vi "UHR-Fleezers Control (host) - 12.7e.vi"() -> ()   [LabVIEW 2012] (continued)
                  frame #11 {
                    n1316 = property on="Load parameters" class="Bool (strict)"("Val(Sgnl)"=TRUE ("Value (Signaling)")) -> ()  [unwired: 2 in, 2 out]
                  }
                }
              }
            }
          }
          frame #9 {
            n1317 = property on="Read Cal" class="Bool (strict)"("Val(Sgnl)"=TRUE ("Value (Signaling)")) -> ()  [unwired: 2 in, 2 out]
          }
          frame #10 {
            n1318 = Wait (ms)(milliseconds to wait=u32 1000) -> ()  [unwired: 1 out]
          }
          frame #11 {
            n1319 = property on="Fish for Tether" class="Bool (strict)"("Val(Sgnl)"=TRUE ("Value (Signaling)")) -> ()  [unwired: 2 in, 2 out]
          }
        }
        n1320 = local write "Cal/Data Acq. Spot"(FALSE ("Cal/Data Acq. Spot")) -> ()
      }
      event "Dump Beads": Value Change {
        n1321 = event-data() -> ()  [unwired: 1 in, 5 out]
        n1322 = flat-sequence {
          tunnel: ["Dump spot flow on?"] -> w1951
          tunnel: [w1962] -> w1952
          tunnel: w1951 -> [w1962]
          tunnel: w1955 -> [w1967]
          tunnel: w1954 -> [w1966]
          tunnel: [w1964] -> w1953
          tunnel: w1952 -> [w1964]
          tunnel: w1953 -> [w1977]
          frame #0 {
            w1956 = FALSE ("Value (Signaling)")
            n1323 = local read "Saving..."() -> (w1958:bool)
            n1324 = local write "Dump Beads"(FALSE ("Dump Beads")) -> ()
            n1325 = property on="Inject Pump 3" class="Bool (strict)"("Val(Sgnl)"=w1956) -> ()  [unwired: 2 in, 2 out]
            n1326 = property on="Inject Pump 1" class="Bool (strict)"("Val(Sgnl)"=w1956) -> ()  [unwired: 2 in, 2 out]
            n1327 = local write "Stop Saving"(w1958) -> ()
          }
          frame #1 {
            w1959 = FALSE ("Fl. Triggered...")
            n1328 = case shown="True" "Dump spot flow on?" {
              frame False {
              }
              frame True {
                n1329 = property on="Sample Channel\nFlow" class="Bool (strict)"("Val(Sgnl)"=TRUE ("Stage Moving")) -> ()  [unwired: 2 in, 2 out]
              }
            }
            n1330 = local write "Fl. Triggered..."(w1959) -> ()
            n1331 = local write "Tether"(w1959) -> ()
            n1332 = property on="Green Laser ON" class="Bool (strict)"("Val(Sgnl)"=w1959) -> ()  [unwired: 2 in, 2 out]
            n1333 = property on="Trap Pos. FB ON" class="Bool (strict)"("Val(Sgnl)"=w1959) -> ()  [unwired: 2 in, 2 out]
            n1334 = property on="Trap Trig. Fl." class="Bool (strict)"("Val(Sgnl)"=w1959) -> ()  [unwired: 2 in, 2 out]
            n1335 = property on="Fl. Triggered..." class="Bool (strict)"("Val(Sgnl)"=w1959) -> ()  [unwired: 2 in, 2 out]
            n1336 = property on="Dip for Protein" class="Bool (strict)"("Val(Sgnl)"=w1959) -> ()  [unwired: 2 in, 2 out]
            n1337 = property on="Pause dwell" class="Bool (strict)"("Val(Sgnl)"=w1959) -> ()  [unwired: 2 in, 2 out]
          }
          frame #2 {
            n1338 = property on="Trap Pos. FB Offset Factor" class="DigNum (strict)"("Val(Sgnl)"=i64 0 ("Value (Signaling)")) -> ()  [unwired: 2 in, 2 out]
          }
          frame #3 {
            n1339 = local read "Saved Stage Positions"() -> (w1968:dbl[][])
            n1340 = local write "Stage Moving"(TRUE ("Stage Moving")) -> ()
            n1341 = Array Subset(array=w1968, index (row)=3 ("index"), length (row)=1 ("length"), index (col)=1 ("index"), length (col)=3 ("length")) -> (w1973:dbl[][])
            n1342 = Reshape Array(w1973, 3 ("dimension size")) -> (w1971:dbl[])
            n1343 = Array To Cluster(array=w1971) -> (cluster=w1970:cluster{"[0]":dbl, "[1]":dbl, "[2]":dbl})
            n1344 = call "Set Stage Position.vi"("Position"=w1970, "error in"=w1966, "VISA resource name in"=w1967) -> ()  [unwired: 3 out]
          }
          frame #4 {
            w1978 = FALSE ("Value (Signaling)")
            n1345 = case shown="True" w1977 {
              frame False {
              }
              frame True {
                n1346 = property on="Sample Channel\nFlow" class="Bool (strict)"("Val(Sgnl)"=FALSE ("Stage Moving")) -> ()  [unwired: 2 in, 2 out]
              }
            }
            n1347 = property on="Trap 1 (ON/OFF)" class="Bool (strict)"("Val(Sgnl)"=w1978) -> ()  [unwired: 2 in, 2 out]
            n1348 = property on="Trap 2 (ON/OFF)" class="Bool (strict)"("Val(Sgnl)"=w1978) -> ()  [unwired: 2 in, 2 out]
            n1349 = call <vilib>:"Beep.vi"() -> ()  [unwired: 3 in, 9 out]
          }
          frame #5 {
            n1350 = property on="Move Cap. 2 (ADig Top)" class="Bool (strict)"("Val(Sgnl)"=TRUE ("Value (Signaling)")) -> ()  [unwired: 2 in, 2 out]
            n1351 = property on="Tab Control" class="TabCtl (strict)"("Val(Sgnl)"=T31."Status" ("Value (Signaling)")) -> ()  [unwired: 2 in, 2 out]
          }
        }
      }
      event "Dip for Protein": Value Change {
        n1352 = event-data() -> ()  [unwired: 1 in, 5 out]
        n1353 = case shown="True" "Dip for Protein" {
          tunnel: w1984 -> [_ w1986]
          tunnel: w1983 -> [_ w1985]
          frame False {
          }
          frame True {
            n1354 = while {
              tunnel: w1986 -> [w1997]
              tunnel: w1985 -> [w1996]
              i -> [w1991]
              stop <- w1993 stop-if-true
              n1355 = Increment(x=w1991) -> (x+1=→"Dip #":i32)
              n1356 = flat-sequence {
                tunnel: w1996 -> [w2008]
                tunnel: w1997 -> [w2009]
                tunnel: [w2009] -> w2001
                tunnel: [w2008] -> w2000
                tunnel: [w2002] -> w1987
                tunnel: [w2014] -> w1995
                tunnel: [w2015] -> w1994
                tunnel: w2001 -> [w2016]
                tunnel: w2000 -> [w2017]
                tunnel: [w2012] -> w1988
                tunnel: w1987 -> [w2012]
                tunnel: [w2025] -> w1999
                tunnel: w1995 -> [w2025]
                tunnel: [w2024] -> w1998
                tunnel: w1994 -> [w2024]
                tunnel: [w2021] -> w1992
                tunnel: [w2020] -> w1989
                tunnel: w1988 -> [w2020]
                tunnel: w1998 -> [w2045]
                tunnel: w1999 -> [w2046]
                tunnel: w1992 -> [w2047]
                tunnel: w1989 -> [w2044]
                tunnel: [w2103] -> w1993
                frame #0 {
                  n1357 = local read "Trap Pos. FB ON"() -> (w2002:bool)
                  n1358 = Compound Arithmetic op=AND("Flow ON\nduring dip?", "FB OFF when \nflow ON", w2002) -> (w2003:bool)
                  n1359 = case shown="True" "Move trap \nbefore dip move?" {
                    frame False {
                    }
                    frame True {
                      n1360 = property on="Trap Delta (MHz)" class="DigNum (strict)"("Val(Sgnl)"="Dipping Delta (MHz)") -> ()  [unwired: 2 in, 2 out]
                    }
                  }
                  n1361 = property on="Green Laser ON" class="Bool (strict)"("Val(Sgnl)"="Green ON\nbefore dip?") -> ()  [unwired: 2 in, 2 out]
                  n1362 = property on="Sample Channel\nFlow" class="Bool (strict)"("Val(Sgnl)"="Flow ON\nduring dip?") -> ()  [unwired: 2 in, 2 out]
                  n1363 = case shown="True" w2003 {
                    frame False {
                    }
                    frame True {
                      n1364 = property on="Trap Pos. FB ON" class="Bool (strict)"("Val(Sgnl)"=FALSE ("Value (Signaling)")) -> ()  [unwired: 2 in, 2 out]
                    }
                  }
                }
                frame #1 {
                  n1365 = local read "Saved Stage Positions"() -> (w2019:dbl[][])
                  n1366 = local write "Cancel dwell"(FALSE ("Cancel dwell")) -> ()
                  n1367 = call "move to saved stage position.vi"("error in"=w2017, "Stage VISA resource name in"=w2016, "Position"="Dip Stage \nPosition", "Saved Stage Positions"=w2019) -> ("VISA resource name out"=w2014:refnum<visa-resource-name>, "error out"=w2015:errorcluster)
                }
                frame #2 {
                  n1368 = node-c288() -> (w2023:T23)  [unwired: 4 in]
                  n1369 = timed-loop {
                    timing: w2023 -> [_]
                    timing-out: [_] -> w2022
                    tunnel: [w2029] -> w2021
                    i -> [w2026]
                    stop <- w2030 stop-if-true
                    n1370 = node-c288() -> ()  [unwired: 1 in, 1 out]
                    n1371 = Greater Or Equal?(x=w2026, y="Dip Duration (s)") -> (x >= y?=w2038:bool)
                    n1372 = local read "Dip for Protein"() -> (w2031:bool)
                    n1373 = local read "Dump Beads"() -> (w2028:bool)
                    n1374 = local read "Cancel dwell"() -> (w2037:bool)
                    n1375 = local read "Pause dwell"() -> (w2034:bool)
                    n1376 = Not(x=w2031) -> (.not. x?=w2036:bool)
                    n1377 = Compound Arithmetic op=OR(w2037, w2038, w2036) -> (w2035:bool)
                    n1378 = Select(t=FALSE, s=w2034, f=w2035) -> (s? t:f=w2032:bool)
                    n1379 = Not(x=w2028) -> (.not. x?=w2027:bool)
                    n1380 = node-c288() -> ()  [unwired: 1 in, 1 out]
                    n1381 = And(x=w2031, y=w2027) -> (x .and. y?=w2029:bool)
                    n1382 = Or(x=w2032, y=w2028) -> (x .or. y?=w2030:bool)
                    "Dip Time (s)" <- w2026
                  }
                  n1383 = node-c288(w2022) -> ()  [unwired: 1 out]
                }
                frame #3 {
                  n1384 = case shown="True" w2047 {
                    tunnel: w2046 -> [_ w2052]
                    tunnel: w2045 -> [_ w2051]
                    tunnel: w2044 -> [_ w2048]
                    frame False {
                    }
                    frame True {
                      n1385 = flat-sequence {
                        tunnel: w2051 -> [w2056]
                        tunnel: w2052 -> [w2057]
                        tunnel: [w2057] -> w2050
                        tunnel: [w2056] -> w2049
                        tunnel: w2048 -> [w2053]
                        tunnel: w2050 -> [w2067]
                        tunnel: w2049 -> [w2066]
                        tunnel: w2048 -> [w2075]
                        frame #0 {
                          n1386 = local read "Sample Channel\nFlow"() -> (w2055:bool)
                          n1387 = case shown="True" w2055 {
                            tunnel: "Flow ON \nduring return\nfrom dip?" -> [w2058 w2061]
                            tunnel: w2053 -> [_ w2060]
                            frame False {
                              n1388 = case shown="True" w2058 {
                                frame False {
                                }
                                frame True {
                                n1389 = property on="Sample Channel\nFlow" class="Bool (strict)"("Val(Sgnl)"=TRUE ("Value (Signaling)")) -> ()  [unwired: 2 in, 2 out]
                                }
                              }
                            }
                            frame True {
                              n1390 = case shown="False" w2061 {
                                tunnel: w2060 -> [w2062 _]
                                frame False {
                                n1391 = property on="Trap Pos. FB ON" class="Bool (strict)"("Val(Sgnl)"=w2062) -> ()  [unwired: 2 in, 2 out]
                                n1392 = property on="Sample Channel\nFlow" class="Bool (strict)"("Val(Sgnl)"=FALSE ("Value (Signaling)")) -> ()  [unwired: 2 in, 2 out]
                                }
                                frame True {
                                }
                              }
                            }
                          }
                        }
                        frame #1 {
                          # "For turning on green laser before stage reaches lower spot"
                          n1393 = case shown="True" "Green ON\nafter start\nreturn?" {
                            frame False {
                            }
                            frame True {
                              n1394 = flat-sequence {
                                frame #0 {
                                n1395 = Multiply(x="Green delay after \nstart return (s)", y=1000.0) -> (x*y=w2072:dbl)
                                n1396 = Wait (ms)(milliseconds to wait=w2072) -> ()  [unwired: 1 out]
                                }
                                frame #1 {
                                n1397 = property on="Green Laser ON" class="Bool (strict)"("Val(Sgnl)"=TRUE ("Value (Signaling)")) -> ()  [unwired: 2 in, 2 out]
                                }
                              }
                            }
                          }
                          n1398 = local read "Saved Stage Positions"() -> (w2070:dbl[][])
                          n1399 = local write "Cancel dwell"(FALSE ("Cancel dwell")) -> ()
                          n1400 = call "move to saved stage position.vi"("error in"=w2066, "Stage VISA resource name in"=w2067, "Position"="Return Stage \nPosition", "Saved Stage Positions"=w2070) -> ("error out"=w2068:errorcluster)  [unwired: 1 out]
                          n1401 = local write "Stage Control Serial Error"(w2068) -> ()
                        }
                        frame #2 {
                          n1402 = property on="Trap Pos. FB ON" class="Bool (strict)"("Val(Sgnl)"=w2075) -> ()  [unwired: 2 in, 2 out]
                          n1403 = case shown="True" "Green ON \nafter return?" {
                            frame False {
                            }
                            frame True {
                              n1404 = property on="Green Laser ON" class="Bool (strict)"("Val(Sgnl)"=TRUE ("Value (Signaling)")) -> ()  [unwired: 2 in, 2 out]
                            }
                          }
                          n1405 = case shown="True" "Move trap after return?" {
                            frame False {
                            }
                            frame True {
                              n1406 = property on="Trap Delta (MHz)" class="DigNum (strict)"("Val(Sgnl)"="Dip Trap Delta 2 (MHz)") -> ()  [unwired: 2 in, 2 out]
                            }
                          }
                          n1407 = case shown="True" "Save data after return?" {
                            frame False {
                            }
                            frame True {
                              n1408 = property on="Start Saving" class="Bool (strict)"("Val(Sgnl)"=TRUE ("Value (Signaling)")) -> ()  [unwired: 2 in, 2 out]
                            }
                          }
                          n1409 = property on="Sample Channel\nFlow" class="Bool (strict)"("Val(Sgnl)"="Flow ON\nduring daq?") -> ()  [unwired: 2 in, 2 out]
                        }
                        frame #3 {
                          n1410 = node-c288() -> (w2084:T23)  [unwired: 4 in]
                          n1411 = timed-loop {
                            timing: w2084 -> [_]
                            timing-out: [_] -> w2083
                            i -> [w2085]
                            stop <- w2087 stop-if-true
                            n1412 = node-c288() -> ()  [unwired: 1 in, 1 out]
                            n1413 = local read "Dump Beads"() -> (w2086:bool)
                            n1414 = Greater Or Equal?(x=w2085, y="Dwell Duration (s)") -> (x >= y?=w2092:bool)
                            n1415 = local read "Dip for Protein"() -> (w2089:bool)
                            n1416 = Not(x=w2089) -> (.not. x?=w2088:bool)
                            n1417 = Compound Arithmetic op=OR(w2092, "Cancel dwell", w2088) -> (w2091:bool)
                            n1418 = node-c288() -> ()  [unwired: 1 in, 1 out]
                            n1419 = Select(t=FALSE, s="Pause dwell", f=w2091) -> (s? t:f=w2094:bool)
                            n1420 = Or(x=w2094, y=w2086) -> (x .or. y?=w2087:bool)
                            "Dwell Time (s)" <- w2085
                          }
                          n1421 = node-c288(w2083) -> ()  [unwired: 1 out]
                        }
                      }
                    }
                  }
                }
                frame #4 {
                  n1422 = local read "Dip for Protein"() -> (w2104:bool)
                  n1423 = local read "Dump Beads"() -> (w2101:bool)
                  n1424 = local write "Cancel dwell"(FALSE ("Cancel dwell")) -> ()
                  n1425 = Not(x=w2104) -> (.not. x?=w2105:bool)
                  n1426 = Not(x="Cont. Repeat Dipping?") -> (.not. x?=w2107:bool)
                  n1427 = Compound Arithmetic op=OR(w2105, w2107, w2101) -> (w2103:bool)
                }
              }
            }
          }
        }
      }
      event "Profile": Value Change {
        n1428 = event-data() -> ()  [unwired: 1 in, 5 out]
        n1429 = flat-sequence {
          tunnel: w2116 -> [w2119]
          tunnel: w2115 -> [w2127]
          tunnel: [w2121] -> w2114
          tunnel: [w2120] -> w2113
          tunnel: [w2118] -> w2111
          tunnel: [w2117] -> w2108
          tunnel: w2114 -> [w2134]
          tunnel: w2113 -> [w2133]
          tunnel: [w2131] -> w2112
          tunnel: w2111 -> [w2132]
          tunnel: [w2130] -> w2110
          tunnel: [w2129] -> w2109
          tunnel: w2108 -> [w2129]
          tunnel: w2112 -> [w2138]
          tunnel: w2110 -> [w2137]
          tunnel: w2109 -> [w2136]
          frame #0 {
            n1430 = call "Read Stage Position.vi"("error in"=w2127, "VISA resource name in"=w2119) -> ("Current Position"=w2117:cluster{dbl, dbl, dbl}, "error out"=w2120:errorcluster, "VISA resource name out"=w2118:refnum<visa-resource-name>)  [unwired: 1 out]
            "Current Position" <- w2117
            n1431 = local write "Stage Control Serial Error"(w2120) -> ()
            n1432 = Unbundle(w2117) -> (w2124:dbl, w2126:dbl, w2122:dbl)
            n1433 = Add(x=w2126, y="Y change (mm)") -> (x+y=w2123:dbl)
            n1434 = Bundle(w2124, w2123, w2122) -> (w2121:cluster{dbl, dbl, dbl})  [unwired: 1 in]
          }
          frame #1 {
            # "move to new position and start saving"
            n1435 = local write "Stage Moving"(TRUE ("Stage Moving")) -> ()
            n1436 = local write "Start Saving"(TRUE ("Start Saving")) -> ()
            n1437 = call "Set Stage Position.vi"("Position"=w2134, "error in"=w2133, "VISA resource name in"=w2132) -> ("error out"=w2130:errorcluster, "VISA resource name out"=w2131:refnum<visa-resource-name>)  [unwired: 1 out]
          }
          frame #2 {
            # "go back to start"
            n1438 = call "Set Stage Position.vi"("Position"=w2136, "error in"=w2137, "VISA resource name in"=w2138) -> ()  [unwired: 3 out]
          }
          frame #3 {
            # "stop saving"
            n1439 = local write "Stop Saving"(TRUE ("Stop Saving")) -> ()
            n1440 = local write "Stage Moving"(FALSE ("Stage Moving")) -> ()
          }
        }
      }
      event "Move to Position 1", "Move to Position 2", "Move to Position 3", "Move to Position 4", "Move to Position 5", "Lower Ch. Cap.": Value Change {
        n1441 = event-data() -> ()  [unwired: 1 in, 5 out]
        n1442 = Or(x="Move to Position 5", y="Lower Ch. Cap.") -> (x .or. y?=w2144:bool)
        n1443 = Build Array("Move to Position 1", "Move to Position 2", "Move to Position 3", "Move to Position 4", w2144) -> (w2147:bool[])
        n1444 = Boolean Array To Number(Boolean array=w2147) -> (number=w2146:u32)
        n1445 = Logarithm Base 2(1:w2146) -> (0:w2145:dbl)
        n1446 = flat-sequence {
          tunnel: w2145 -> [w2156]
          tunnel: w2142 -> [w2154]
          tunnel: w2141 -> [w2153]
          frame #0 {
            n1447 = local read "Saved Stage Positions"() -> (w2164:dbl[][])
            n1448 = Array Subset(array=w2164, index (row)=w2156, length (row)=1 ("length"), index (col)=1 ("index"), length (col)=3 ("length")) -> (w2161:dbl[][])
            n1449 = Reshape Array(w2161, 3 ("dimension size")) -> (w2159:dbl[])
            n1450 = Array To Cluster(array=w2159) -> (cluster=w2158:cluster{"[0]":dbl, "[1]":dbl, "[2]":dbl})
            n1451 = call "Set Stage Position.vi"("Position"=w2158, "error in"=w2153, "VISA resource name in"=w2154) -> ("error out"=w2157:errorcluster)  [unwired: 2 out]
            n1452 = local write "Stage Moving"(TRUE ("Stage Moving")) -> ()
            n1453 = local write "Stage Control Serial Error"(w2157) -> ()
          }
          frame #1 {
            n1454 = local write "Stage Moving"(FALSE ("Stage Moving")) -> ()
            n1455 = call <vilib>:"Beep.vi"() -> ()  [unwired: 3 in, 9 out]
          }
        }
      }
      event "Got ADig bead": Value Change {
        n1456 = event-data() -> ()  [unwired: 1 in, 5 out]
        n1457 = flat-sequence {
          frame #0 {
            n1458 = local read "Cap 1 Samp Flow ON"() -> (w2168:bool)
            n1459 = case shown="True" w2168 {
              frame False {
              }
              frame True {
                n1460 = property on="Sample Channel\nFlow" class="Bool (strict)"("Val(Sgnl)"=TRUE ("Value (Signaling)")) -> ()  [unwired: 2 in, 2 out]
              }
            }
          }
          frame #1 {
            n1461 = property on="Inject Pump 3" class="Bool (strict)"("Val(Sgnl)"=FALSE ("Value (Signaling)")) -> ()  [unwired: 2 in, 2 out]
          }
          frame #2 {
            n1462 = property on="Move Cap. 1 (DNA Bottom)" class="Bool (strict)"("Val(Sgnl)"=TRUE ("Value (Signaling)")) -> ()  [unwired: 2 in, 2 out]
          }
        }
      }
      event "Force FB Data\nScript": Value Change {
        n1463 = event-data() -> ()  [unwired: 1 in, 5 out]
        n1464 = flat-sequence {
          tunnel: w2177 -> [w2181]
          tunnel: w2178 -> [w2182]
          tunnel: [w2182] -> w2173
          tunnel: [w2181] -> w2172
          tunnel: w2173 -> [w2185]
          tunnel: w2172 -> [w2184]
          tunnel: ["Trap Trig Fl."] -> w2174
          tunnel: [w2210] -> w2175
          tunnel: w2174 -> [w2210]
          tunnel: [w2214] -> w2176
          tunnel: w2175 -> [w2214]
          tunnel: w2176 -> [w2216]
          frame #0 {
            n1465 = property on="Trap Delta (MHz)" class="DigNum (strict)"("Val(Sgnl)"="Trap Delta Before Moving") -> ()  [unwired: 2 in, 2 out]
          }
          frame #1 {
            n1466 = local read "Saved Stage Positions"() -> (w2187:dbl[][])
            n1467 = local write "FB Trap Pos Offset"(0.0 ("FB Trap Pos Offset")) -> ()
            n1468 = property on="Trap Pos. FB Offset Factor" class="DigNum (strict)"("Val(Sgnl)"=i64 0 ("Value (Signaling)")) -> ()  [unwired: 2 in, 2 out]
            n1469 = local write "Stage Moving"(TRUE ("Stage Moving")) -> ()
            n1470 = call "move to saved stage position.vi"("error in"=w2184, "Stage VISA resource name in"=w2185, "Position"="Stage Position To Establish FB", "Saved Stage Positions"=w2187) -> ("error out"=w2183:errorcluster)  [unwired: 1 out]
            n1471 = local write "Stage Control Serial Error"(w2183) -> ()
          }
          frame #2 {
            n1472 = call <vilib>:"Beep.vi"() -> ()  [unwired: 3 in, 9 out]
            n1473 = Multiply(x="Wait (s)", y=u32 1000 ("milliseconds to wait")) -> (x*y=w2194:u32)
            n1474 = property on="Trap Delta (MHz)" class="DigNum (strict)"("Val(Sgnl)"="Starting \nTrap Delta (MHz)") -> ()  [unwired: 2 in, 2 out]
            n1475 = local write "Stage Moving"(FALSE ("Stage Moving")) -> ()
            n1476 = Wait (ms)(milliseconds to wait=w2194) -> ()  [unwired: 1 out]
            n1477 = property on="Tab Control 2" class="TabCtl (strict)"("Val(Sgnl)"=T6."Feedback on Trap Position" ("Value (Signaling)")) -> ()  [unwired: 2 in, 2 out]
            n1478 = property on="Tab Control" class="TabCtl (strict)"("Val(Sgnl)"=T32."Trap Control (RF)" ("Value (Signaling)")) -> ()  [unwired: 2 in, 2 out]
          }
          frame #3 {
            n1479 = property on="Set Reading to\nSetpoint" class="Bool (strict)"("Val(Sgnl)"=TRUE ("Value (Signaling)")) -> ()  [unwired: 2 in, 2 out]
            n1480 = Wait (ms)(milliseconds to wait=u32 500) -> ()  [unwired: 1 out]
          }
          frame #4 {
            n1481 = property on="Trap Pos. FB ON" class="Bool (strict)"("Val(Sgnl)"=TRUE ("Value (Signaling)")) -> ()  [unwired: 2 in, 2 out]
            n1482 = Wait (ms)(milliseconds to wait=u32 250) -> ()  [unwired: 1 out]
          }
          frame #5 {
            n1483 = case shown="False" "Trap Trig Fl." {
              frame False {
                n1484 = case shown="True" "Green ON after FB ON?" {
                  selector: "Green ON after FB ON?" -> [_ w2209]
                  frame False {
                  }
                  frame True {
                    n1485 = property on="Green Laser ON" class="Bool (strict)"("Val(Sgnl)"=w2209) -> ()  [unwired: 2 in, 2 out]
                  }
                }
              }
              frame True {
              }
            }
            n1486 = case shown="True" "Remove Action Offset" {
              tunnel: TRUE ("Value (Signaling)") -> [w2206 w2207]
              frame False {
                n1487 = property on="Remove Unwinding Offset" class="Bool (strict)"("Val(Sgnl)"=w2206) -> ()  [unwired: 2 in, 2 out]
              }
              frame True {
                n1488 = property on="Remove Action Offset" class="Bool (strict)"("Val(Sgnl)"=w2207) -> ()  [unwired: 2 in, 2 out]
              }
            }
            n1489 = Wait (ms)(milliseconds to wait=u32 250) -> ()  [unwired: 1 out]
          }
          frame #6 {
            n1490 = property on="Start Saving" class="Bool (strict)"("Val(Sgnl)"=TRUE ("Value (Signaling)")) -> ()  [unwired: 2 in, 2 out]
            n1491 = Wait (ms)(milliseconds to wait=u32 5000) -> ()  [unwired: 1 out]
          }
          frame #7 {
            w2213 = TRUE ("Value (Signaling)")
            n1492 = property on="Rem fb disp offset" class="Bool (strict)"("Val(Sgnl)"=w2213) -> ()  [unwired: 2 in, 2 out]
            n1493 = property on="Remove Offset" class="Bool (strict)"("Val(Sgnl)"=w2213) -> ()  [unwired: 2 in, 2 out]
            n1494 = Wait (ms)(milliseconds to wait=u32 100) -> ()  [unwired: 1 out]
          }
          frame #8 {
            n1495 = case shown="True" w2216 {
              frame False {
              }
              frame True {
                n1496 = local write "Trap Trig. Fl."(TRUE ("Value (Signaling)")) -> ()
              }
            }
          }
          frame #9 {
            n1497 = case shown="True" "Start dipping after?" {
              frame False {
              }
              frame True {
                n1498 = flat-sequence {
                  frame #0 {
                    n1499 = Multiply(x="Delay before dipping (s)", y=1000.0) -> (x*y=w2220:dbl)
                    n1500 = Wait (ms)(milliseconds to wait=w2220) -> ()  [unwired: 1 out]
                  }
                  frame #1 {
                    n1501 = property on="Dip for Protein" class="Bool (strict)"("Val(Sgnl)"=TRUE ("Value (Signaling)")) -> ()  [unwired: 2 in, 2 out]
                    n1502 = local write "Scripts"(T1."Dipping" ("Scripts")) -> ()
                  }
                }
              }
            }
          }
        }
      }
      event "Fixed Traps Data\nScript": Value Change {
        n1503 = event-data() -> ()  [unwired: 1 in, 5 out]
        n1504 = flat-sequence {
          frame #0 {
            n1505 = case shown="True" "Green ON" {
              frame False {
              }
              frame True {
                n1506 = property on="Green Laser ON" class="Bool (strict)"("Val(Sgnl)"=TRUE) -> ()  [unwired: 2 in, 2 out]
              }
            }
            n1507 = local write "Offset (nm)"(0.0 ("Offset (nm)")) -> ()
            n1508 = property on="Sample Channel\nFlow" class="Bool (strict)"("Val(Sgnl)"=FALSE ("Value (Signaling)")) -> ()  [unwired: 2 in, 2 out]
            n1509 = property on="Trap Delta (MHz)" class="DigNum (strict)"("Val(Sgnl)"="Fixed Traps Trap Delta (MHz)") -> ()  [unwired: 2 in, 2 out]
          }
          frame #1 {
            n1510 = Wait (ms)(milliseconds to wait=u32 1000) -> ()  [unwired: 1 out]
          }
          frame #2 {
            n1511 = local write "Start Saving"(TRUE ("Start Saving")) -> ()
          }
          frame #3 {
            n1512 = local read "Bead Sep. Int. Time (s)"() -> (w2231:dbl)
            n1513 = Multiply(x=w2231, y=1000.0) -> (x*y=w2233:dbl)
            n1514 = Wait (ms)(milliseconds to wait=w2233) -> ()  [unwired: 1 out]
          }
          frame #4 {
            n1515 = property on="Remove Offset" class="Bool (strict)"("Val(Sgnl)"=TRUE ("Value (Signaling)")) -> ()  [unwired: 2 in, 2 out]
          }
          frame #5 {
            n1516 = property on="Dip for Protein" class="Bool (strict)"("Val(Sgnl)"="Start dipping after?") -> ()  [unwired: 2 in, 2 out]
          }
        }
      }
      event "Got DNA bead": Value Change {
        n1517 = event-data() -> ()  [unwired: 1 in, 5 out]
        n1518 = flat-sequence {
          frame #0 {
            n1519 = local read "Daq spot flow on"() -> (w2238:bool)
            n1520 = case shown="True" w2238 {
              frame False {
              }
              frame True {
                n1521 = property on="Sample Channel\nFlow" class="Bool (strict)"("Val(Sgnl)"=TRUE ("Value (Signaling)")) -> ()  [unwired: 2 in, 2 out]
              }
            }
            n1522 = property on="Got DNA bead" class="Bool"("Key Focus"=FALSE) -> ()  [unwired: 2 in, 2 out]
          }
          frame #1 {
            n1523 = property on="Inject Pump 1" class="Bool (strict)"("Val(Sgnl)"=FALSE ("Value (Signaling)")) -> ()  [unwired: 2 in, 2 out]
          }
          frame #2 {
            n1524 = property on="Cal/Data Acq. Spot" class="Bool (strict)"("Val(Sgnl)"=TRUE ("Value (Signaling)")) -> ()  [unwired: 2 in, 2 out]
          }
        }
      }
      event "Take Stepping Data": Value Change {
        n1525 = event-data() -> ()  [unwired: 1 in, 5 out]
        n1526 = local read "Save ave N"() -> (w2250:dbl)
        n1527 = flat-sequence {
          tunnel: w2250 -> [w2252]
          tunnel: [w2252] -> w2245
          tunnel: [w2254] -> w2246
          tunnel: w2245 -> [w2254]
          tunnel: [w2256] -> w2247
          tunnel: w2246 -> [w2256]
          tunnel: [w2259] -> w2248
          tunnel: w2247 -> [w2259]
          tunnel: [w2261] -> w2249
          tunnel: w2248 -> [w2261]
          tunnel: [w2263] -> w2243
          tunnel: w2249 -> [w2263]
          tunnel: w2243 -> [w2266]
          tunnel: [w2266] -> w2242
          tunnel: w2242 -> [w2267]
          tunnel: [w2267] -> w2244
          tunnel: w2244 -> [w2273]
          frame #0 {
            n1528 = property on="Save ave N" class="DigNum (strict)"("Val(Sgnl)"="Save ave factor") -> ()  [unwired: 2 in, 2 out]
          }
          frame #1 {
            n1529 = Wait (ms)(milliseconds to wait=u32 100) -> ()  [unwired: 1 out]
          }
          frame #2 {
            n1530 = local read "Offset 2 Start (MHz)"() -> (w2258:dbl)
            n1531 = property on="Saved AOD Raster Scan Parameter Sets" class="Arr (strict)"("Index Values"=u32[] [2]) -> ()  [unwired: 2 in, 2 out]
            n1532 = property on="Trap Delta (MHz)" class="DigNum (strict)"("Val(Sgnl)"=w2258) -> ()  [unwired: 2 in, 2 out]
          }
          frame #3 {
            n1533 = property on="Load parameters" class="Bool (strict)"("Val(Sgnl)"=TRUE ("Value (Signaling)")) -> ()  [unwired: 2 in, 2 out]
          }
          frame #4 {
            n1534 = Wait (ms)(milliseconds to wait=u32 100) -> ()  [unwired: 1 out]
          }
          frame #5 {
            n1535 = property on="Trap Raster Scan" class="Bool (strict)"("Val(Sgnl)"=TRUE ("Value (Signaling)")) -> ()  [unwired: 2 in, 2 out]
          }
          frame #6 {
            n1536 = Wait (ms)(milliseconds to wait=u32 1000) -> ()  [unwired: 1 out]
          }
          frame #7 {
            n1537 = while {
              stop <- w2270 stop-if-true
              n1538 = local read "Raster Scanning..."() -> (w2272:bool)
              n1539 = local read "Saving..."() -> (w2271:bool)
              n1540 = Not(x=w2271) -> (.not. x?=w2268:bool)
              n1541 = Not(x=w2272) -> (.not. x?=w2269:bool)
              n1542 = And(x=w2269, y=w2268) -> (x .and. y?=w2270:bool)
            }
          }
          frame #8 {
            n1543 = property on="Save ave N" class="DigNum (strict)"("Val(Sgnl)"=w2273) -> ()  [unwired: 2 in, 2 out]
          }
        }
      }
      event "Step Size (nm)": Value Change {
        n1544 = event-data() -> ()  [unwired: 1 in, 5 out]
        n1545 = flat-sequence {
          frame #0 {
            n1546 = property on="Saved AOD Raster Scan Parameter Sets" class="Arr (strict)"("Index Values"=u32[] [1]) -> ()  [unwired: 2 in, 2 out]
          }
          frame #1 {
            n1547 = Multiply(x="N Steps", y="Step Size (nm)") -> (x*y=w2275:dbl)
            n1548 = property on="Scan Speed AOD (nm/s) 2" class="DigNum (strict)"("Value"="Step Size (nm)") -> ()  [unwired: 2 in, 2 out]
            n1549 = property on="Step Size AOD (nm) 2" class="DigNum (strict)"("Value"="Step Size (nm)") -> ()  [unwired: 2 in, 2 out]
            n1550 = property on="Scan Range AOD (nm) 2" class="DigNum (strict)"("Value"=w2275) -> ()  [unwired: 2 in, 2 out]
          }
        }
      }
      event "Take Detection Laser\nImage": Value Change {
        n1551 = event-data() -> ()  [unwired: 1 in, 5 out]
        n1552 = flat-sequence {
          tunnel: [w2303] -> w2293
          tunnel: [w2302] -> w2286
          tunnel: [w2301] -> w2278
          tunnel: [w2306] -> w2294
          tunnel: w2293 -> [w2306]
          tunnel: [w2305] -> w2287
          tunnel: w2286 -> [w2305]
          tunnel: [w2304] -> w2279
          tunnel: w2278 -> [w2304]
          tunnel: [w2310] -> w2295
          tunnel: w2294 -> [w2310]
          tunnel: [w2309] -> w2288
          tunnel: w2287 -> [w2309]
          tunnel: [w2308] -> w2280
          tunnel: w2279 -> [w2308]
          tunnel: [w2316] -> w2296
          tunnel: w2295 -> [w2316]
          tunnel: [w2315] -> w2289
          tunnel: w2288 -> [w2315]
          tunnel: [w2314] -> w2281
          tunnel: w2280 -> [w2314]
          tunnel: [w2320] -> w2297
          tunnel: w2296 -> [w2320]
          tunnel: [w2319] -> w2290
          tunnel: w2289 -> [w2319]
          tunnel: [w2318] -> w2282
          tunnel: w2281 -> [w2318]
          tunnel: [w2324] -> w2298
          tunnel: w2297 -> [w2324]
          tunnel: [w2323] -> w2291
          tunnel: w2290 -> [w2323]
          tunnel: [w2322] -> w2283
          tunnel: w2282 -> [w2322]
          tunnel: [w2328] -> w2299
          tunnel: w2298 -> [w2328]
          tunnel: [w2327] -> w2292
          tunnel: w2291 -> [w2327]
          tunnel: [w2326] -> w2284
          tunnel: w2283 -> [w2326]
          tunnel: w2299 -> [w2334]
          tunnel: w2292 -> [w2333]
          tunnel: [w2331] -> w2285
          tunnel: w2284 -> [w2331]
          tunnel: w2285 -> [w2335]
          frame #0 {
            n1553 = local read "Laser interlacing mode"() -> (w2302:enum32{"Laser ON", "Laser OFF", "Interlace"})
            n1554 = local read "Green FB On/Off"() -> (w2301:bool)
            n1555 = local read "Green Laser ON"() -> (w2303:bool)
          }
          frame #1 {
            n1556 = property on="Green FB On/Off" class="Bool (strict)"("Val(Sgnl)"=FALSE ("Value (Signaling)")) -> ()  [unwired: 2 in, 2 out]
          }
          frame #2 {
            n1557 = property on="Green Laser ON" class="Bool (strict)"("Val(Sgnl)"=TRUE ("Value (Signaling)")) -> ()  [unwired: 2 in, 2 out]
            n1558 = property on="Flip Green Filter" class="Bool (strict)"("Val(Sgnl)"=TRUE ("Value (Signaling)")) -> ()  [unwired: 2 in, 2 out]
            n1559 = property on="Laser interlacing mode" class="RadioBtnsControl (strict)"("Val(Sgnl)"=enum32{"Laser ON", "Laser OFF", "Interlace"}."Laser ON" ("Value (Signaling)")) -> ()  [unwired: 2 in, 2 out]
          }
          frame #3 {
            n1560 = Wait (ms)(milliseconds to wait=u32 500) -> ()  [unwired: 1 out]
          }
          frame #4 {
            n1561 = property on="Confocal Image" class="Bool (strict)"("Val(Sgnl)"=TRUE ("Value (Signaling)")) -> ()  [unwired: 2 in, 2 out]
          }
          frame #5 {
            n1562 = Wait (ms)(milliseconds to wait=u32 2000) -> ()  [unwired: 1 out]
          }
          frame #6 {
            n1563 = while {
              stop <- w2329 stop-if-true
              n1564 = local read "Saving..."() -> (w2330:bool)
              n1565 = Not(x=w2330) -> (.not. x?=w2329:bool)
            }
          }
          frame #7 {
            n1566 = property on="Flip Green Filter" class="Bool (strict)"("Val(Sgnl)"=TRUE ("Value (Signaling)")) -> ()  [unwired: 2 in, 2 out]
            n1567 = property on="Green Laser ON" class="Bool (strict)"("Val(Sgnl)"=w2334) -> ()  [unwired: 2 in, 2 out]
            n1568 = property on="Laser interlacing mode" class="RadioBtnsControl (strict)"("Val(Sgnl)"=w2333) -> ()  [unwired: 2 in, 2 out]
          }
          frame #8 {
            n1569 = property on="Green FB On/Off" class="Bool (strict)"("Val(Sgnl)"=w2335) -> ()  [unwired: 2 in, 2 out]
          }
        }
      }
      event "Move in a Circle": Value Change {
        w2337 = dbl[] []
        # "converting distance (d) to angle (a)\na=arcsin(d/2r)"
        # "radius"
        # "radius"
        # "T1 Y"
        # "T1 X"
        n1570 = event-data() -> ()  [unwired: 1 in, 5 out]
        n1571 = local read "BD 1 Frequency 1 (MHz)"() -> (w2345:dbl)
        n1572 = local read "BD 2 Frequency 1 (MHz)"() -> (w2344:dbl)
        n1573 = local read "BD 1 Frequency 2 (MHz)"() -> (w2343:dbl)
        n1574 = local read "BD 2 Frequency 2 (MHz)"() -> (w2342:dbl)
        n1575 = Subtract(x=w2344, y="Center Y Frequency (MHz)") -> (x-y=w2349:dbl)
        n1576 = Absolute Value(x=w2349) -> (abs(x)=w2340:dbl)
        n1577 = flat-sequence {
          tunnel: w2340 -> [w2352]
          tunnel: [w2352] -> w2339
          frame #0 {
            n1578 = local write "Radius (MHz)"(w2352) -> ()
          }
        }
        n1579 = node-c288("Time step (ms)") -> (w2351:T23)  [unwired: 3 in]
        n1580 = timed-loop {
          timing: w2351 -> [_]
          timing-out: [_] -> w2350
          tunnel: w2345 -> [w2443]
          tunnel: w2344 -> [_]
          tunnel: w2343 -> [w2447]
          tunnel: w2342 -> [_]
          tunnel: "Center Y Frequency (MHz)" -> [w2436]
          shift-right: [w2397] -> _
          shift-left: w2337 -> [w2404]
          shift-right: [w2395] -> _
          shift-left: w2337 -> [w2403]
          shift-right: [w2388] -> _
          shift-left: w2337 -> [w2401]
          shift-right: [w2386] -> _
          shift-left: w2337 -> [w2400]
          tunnel: "Move in a Circle" -> [_]
          tunnel: ["Back to start on finish?"] -> w2341
          tunnel: w2339 -> [_]
          tunnel: w2338 -> [w2418]
          tunnel: w2337 -> [w2399]
          shift-right: [w2370] -> _
          shift-left: 0.0 -> [w2368]
          i -> [w2377]
          stop <- w2441 stop-if-true
          w2385 = 0 ("index")
          w2406 = 1 ("dimension size")
          # "Keep phase within\n2pi so errors don't \nbuild"
          # "Accumulated\nphase"
          # "Current phase"
          # "Trap 2"
          # "Trap 1"
          # "ignore if N = 0"
          # "r"
          # "r"
          # "r"
          # "r"
          # "\"omega*t\""
          # "Trap 2"
          # "Trap separation (radians)"
          # "Trap 1"
          # "Offset (starts\n at bottom of\n the circle)"
          # "omega"
          n1581 = node-c288() -> (w2454:i64)  [unwired: 1 in]
          n1582 = Divide(x=w2454, y=1000) -> (x/y=w2373:dbl)
          n1583 = Divide(x="2D Motion Trap Separation (MHz)", y="Radius (MHz)") -> (x/y=w2428:dbl)
          n1584 = Negate(x=w2373) -> (-x=w2372:dbl)
          n1585 = Divide(x="Trap 2 phase shift (deg)", y=360.0) -> (x/y=w2419:dbl)
          n1586 = Inverse Sine(1:w2428) -> (0:w2364:dbl)
          n1587 = Multiply(x=6.283185307179586, y=w2419) -> (x*y=w2365:dbl)
          n1588 = Multiply(x=6.283185307179586, y="2D Motion Frequency (Hz)") -> (x*y=w2376:dbl)
          n1589 = Select(t=w2373, s="Counterclockwise/Clockwise", f=w2372) -> (s? t:f=w2375:dbl)
          n1590 = Multiply(x=w2376, y=w2375) -> (x*y=w2366:dbl)
          n1591 = Select(t=w2364, s="Trap shift\nmethod", f=w2365) -> (s? t:f=w2363:dbl)
          n1592 = Add(x=w2366, y=w2368) -> (x+y=w2369:dbl)
          n1593 = Add(x=w2369, y=w2363) -> (x+y=w2425:dbl)
          n1594 = Add(x=w2369, y=1.5707963267948966) -> (x+y=w2374:dbl)
          n1595 = Add(x=w2425, y=1.5707963267948966) -> (x+y=w2438:dbl)
          n1596 = Cosine(x=w2374) -> (cos(x)=w2452:dbl)
          n1597 = Sine(x=w2374) -> (sin(x)=w2451:dbl)
          n1598 = Multiply(x=w2452, y="Radius (MHz)") -> (x*y=w2445:dbl)
          n1599 = Cosine(x=w2438) -> (cos(x)=w2450:dbl)
          n1600 = Sine(x=w2438) -> (sin(x)=w2449:dbl)
          n1601 = Multiply(x=w2451, y="Radius (MHz)") -> (x*y=w2444:dbl)
          n1602 = Multiply(x=w2450, y="Radius (MHz)") -> (x*y=w2448:dbl)
          n1603 = Multiply(x=w2449, y="Radius (MHz)") -> (x*y=w2446:dbl)
          n1604 = Add(x=w2445, y=w2443) -> (x+y=w2394:dbl)
          n1605 = Add(x=w2444, y=w2436) -> (x+y=w2392:dbl)
          n1606 = Greater Or Equal?(x=w2377, y="N steps then stop") -> (x >= y?=w2435:bool)
          n1607 = Add(x=w2448, y=w2447) -> (x+y=w2383:dbl)
          n1608 = Add(x=w2446, y=w2436) -> (x+y=w2381:dbl)
          n1609 = Not Equal To 0?(x="N steps then stop") -> (x != 0?=w2431:bool)
          n1610 = And(x=w2435, y=w2431) -> (x .and. y?=w2432:bool)
          n1611 = local read "Trap 1 sum mean"() -> (w2415:dbl)
          n1612 = local read "Stop All"() -> (w2440:bool)
          n1613 = local write "BD 1 Frequency 1 (MHz)"(w2394) -> ()
          n1614 = local write "BD 2 Frequency 1 (MHz)"(w2392) -> ()
          n1615 = local write "BD 1 Frequency 2 (MHz)"(w2383) -> ()
          n1616 = local write "BD 2 Frequency 2 (MHz)"(w2381) -> ()
          n1617 = Select(t=w2377, s="test", f=w2415) -> (s? t:f=→"Waveform Chart":dbl)
          n1618 = Compound Arithmetic op=OR(w2440, "Stop Moving", w2432) -> (w2441:bool)
          n1619 = local read "BD 1 Frequency 3 (MHz)"() -> (w2424:dbl)
          n1620 = local read "BD 2 Frequency 3 (MHz)"() -> (w2423:dbl)
          n1621 = Select(t=w2399, s="Reset graph", f=w2400) -> (s? t:f=w2380:dbl[])
          n1622 = Select(t=w2399, s="Reset graph", f=w2401) -> (s? t:f=w2382:dbl[])
          n1623 = Select(t=w2399, s="Reset graph", f=w2403) -> (s? t:f=w2391:dbl[])
          n1624 = Select(t=w2399, s="Reset graph", f=w2404) -> (s? t:f=w2393:dbl[])
          n1625 = Initialize Array(w2381, w2406) -> (w2407:dbl[])
          n1626 = Initialize Array(w2392, w2406) -> (w2410:dbl[])
          n1627 = Initialize Array(w2383, w2406) -> (w2408:dbl[])
          n1628 = Initialize Array(w2394, w2406) -> (w2411:dbl[])
          n1629 = local read "Y RF Frequency Limits (MHz)"() -> (w2421:T16)
          n1630 = local read "X RF Frequency Limits (MHz)"() -> (w2422:T16)
          n1631 = call "set RF board frequency - interlace.vi"("Board 2 Frequency Limits"=w2421, "Board 1 Frequency Limits"=w2422, "FPGA VI Reference In"=w2418, "Board 2 Frequency 3 (MHz)"=w2423, "Board 1 Frequency 3 (MHz)"=w2424, "Board 2 Frequency 2 (MHz)"=w2381, "Board 2 Frequency 1 (MHz)"=w2392, "Board 1 Frequency 2 (MHz)"=w2383, "Board 1 Frequency 1  (MHz)"=w2394) -> ()  [unwired: 1 in, 2 out]
          n1632 = Bundle(w2408, w2407) -> (w2379:cluster{dbl[], dbl[]})  [unwired: 1 in]
          n1633 = Bundle(w2411, w2410) -> (w2409:cluster{dbl[], dbl[]})  [unwired: 1 in]
          n1634 = Build Array (concatenate)(w2394, w2393) -> (w2398:dbl[])
          n1635 = Build Array (concatenate)(w2392, w2391) -> (w2396:dbl[])
          n1636 = Build Array (concatenate)(w2383, w2382) -> (w2389:dbl[])
          n1637 = Build Array (concatenate)(w2381, w2380) -> (w2387:dbl[])
          n1638 = Bundle(w2398, w2396) -> (w2378:cluster{dbl[], dbl[]})  [unwired: 1 in]
          n1639 = Bundle(w2389, w2387) -> (w2405:cluster{dbl[], dbl[]})  [unwired: 1 in]
          n1640 = Build Array(w2409, w2379, w2378, w2405) -> (→"Trap trajectories":cluster{dbl[], dbl[]}[])
          n1641 = case "To pause the process" shown="True" "Pause rotation" {
            frame False {
            }
            frame True {
              n1642 = while {
                stop <- w2457 stop-if-true
                n1643 = local read "Pause rotation"() -> (w2458:bool)
                n1644 = Wait (ms)(milliseconds to wait=u32 10) -> ()  [unwired: 1 out]
                n1645 = Not(x=w2458) -> (.not. x?=w2457:bool)
              }
            }
          }
          n1646 = Decrement(x="N steps to plot") -> (x-1=w2384:i32)
          n1647 = Array Subset(array=w2396, index=w2385, length=w2384) -> (w2395:dbl[])
          n1648 = Array Subset(array=w2398, index=w2385, length=w2384) -> (w2397:dbl[])
          n1649 = Array Subset(array=w2389, index=w2385, length=w2384) -> (w2388:dbl[])
          n1650 = Array Subset(array=w2387, index=w2385, length=w2384) -> (w2386:dbl[])
          n1651 = Quotient & Remainder(x=w2369, y=6.283185307179586) -> (x-y*floor(x/y)=w2370:dbl)  [unwired: 1 out]
          n1652 = node-c288() -> ()  [unwired: 1 in, 1 out]
        }
        n1653 = node-c288(w2350) -> ()  [unwired: 1 out]
        n1654 = case shown="True" w2341 {
          tunnel: w2345 -> [_ w2356]
          tunnel: w2344 -> [_ w2355]
          tunnel: w2343 -> [_ w2354]
          tunnel: w2342 -> [_ w2353]
          frame False {
          }
          frame True {
            n1655 = flat-sequence {
              tunnel: w2356 -> [w2360]
              tunnel: w2355 -> [w2359]
              tunnel: w2354 -> [w2358]
              tunnel: w2353 -> [w2357]
              frame #0 {
                n1656 = local write "BD 1 Frequency 1 (MHz)"(w2360) -> ()
                n1657 = local write "BD 2 Frequency 1 (MHz)"(w2359) -> ()
                n1658 = local write "BD 1 Frequency 2 (MHz)"(w2358) -> ()
                n1659 = local write "BD 2 Frequency 2 (MHz)"(w2357) -> ()
              }
              frame #1 {
                n1660 = property on="Update all trap values" class="Bool (strict)"("Val(Sgnl)"=TRUE ("Value (Signaling)")) -> ()  [unwired: 2 in, 2 out]
              }
            }
          }
        }
      }
      event "Stop All": Value Change {
        # "Stopping blue laser before shutting off program"
        n1661 = event-data() -> ()  [unwired: 1 in, 5 out]
        n1662 = local read "Delay (ms)"() -> (w2468:i32)
        n1663 = call "serial write macro.vi"("String"="l0", "Delay (ms)"=w2468, "VISA resource name"=w2471) -> ("read buffer"=w2466:string, "error out"=w2467:errorcluster, "VISA resource name out"=w2470:refnum<visa-resource-name>)
        n1664 = local write "read blue buffer"(w2466) -> ()
        n1665 = local write "Blue Error Out"(w2467) -> ()
        n1666 = VISA Close(VISA resource name=w2470) -> ()  [unwired: 1 in, 1 out]
        n1667 = local read "Stop All"() -> (w2472:bool)
      }
    }
    n1668 = node-c288() -> ()  [unwired: 1 in, 1 out]
  }
  n1669 = timed-loop "Oscillate Trap/AOM (fishing, conjugate plane alignment)" {
    tunnel: [w2474] -> w69
    timing: w64 -> [_]
    timing-out: [_] -> w63
    tunnel: w5 -> [w2473]
    stop <- w2474 stop-if-true
    n1670 = node-c288() -> ()  [unwired: 2 out]
    n1671 = event shown="[0] \"Oscillate Set 1\", \"Fish for Tether\": Value Change" {
      selector: _ -> [_ _ _]
      dyn-events: _ -> [_ _ _]
      timeout: _ -> [_ _ _]
      tunnel: [FALSE ("Stop All") _ w3079] -> w2474
      tunnel: w2473 -> [w2477 _ _]
      event "Oscillate Set 1", "Fish for Tether": Value Change {
        n1672 = event-data() -> ()  [unwired: 6 out]
        n1673 = local read "Oscillate Set 1"() -> (w2481:bool)
        n1674 = Or(x=w2481, y="Fish for Tether") -> (x .or. y?=w2479:bool)
        n1675 = case shown="True" w2479 {
          tunnel: "Fish for Tether" -> [_ w2484]
          tunnel: w2477 -> [_ w2482]
          frame False {
          }
          frame True {
            n1676 = case shown="True" w2484 {
              selector: w2484 -> [w2487 w2493]
              tunnel: [w2487 w2493] -> w2483
              frame False {
              }
              frame True {
                n1677 = local write "Scan axis 2"(TRUE) -> ()
                n1678 = local write "Tether"(FALSE ("Tether")) -> ()
                n1679 = local read "Flow ON during cal?"() -> (w2488:bool)
                n1680 = property on="Trap Delta (MHz)" class="DigNum (strict)"("Val(Sgnl)"="Furthest Delta (MHz)") -> ()  [unwired: 2 in, 2 out]
                n1681 = Or(x="Flow ON during \nfishing?", y=w2488) -> (x .or. y?=w2489:bool)
                n1682 = Wait (ms)(milliseconds to wait=u32 500) -> ()  [unwired: 1 out]
                n1683 = property on="Sample Channel\nFlow" class="Bool (strict)"("Val(Sgnl)"=w2489) -> ()  [unwired: 2 in, 2 out]
              }
            }
            n1684 = node-c288() -> (w2486:T23)  [unwired: 1 in, 3 out]
            n1685 = timed-loop "Oscillate AOD" {
              timing: w2486 -> [_]
              timing-out: [_] -> w2485
              tunnel: w2483 -> [w2497]
              tunnel: w2482 -> [w2496]
              i -> [w2505]
              stop <- w2503 stop-if-true
              n1686 = node-c288() -> (w2504:i64)  [unwired: 1 out]
              n1687 = flat-sequence {
                tunnel: w2505 -> [w2532]
                tunnel: w2504 -> [w2531]
                tunnel: w2497 -> [w2515]
                tunnel: [w2515] -> w2502
                tunnel: [w2514] -> w2501
                tunnel: [w2513] -> w2500
                tunnel: [w2510] -> w2498
                tunnel: w2496 -> [w2506]
                tunnel: w2502 -> [w2577]
                tunnel: w2501 -> [w2575]
                tunnel: w2500 -> [w2574]
                tunnel: [w2573] -> w2499
                tunnel: w2498 -> [w2572]
                tunnel: [w2649] -> w2503
                tunnel: w2499 -> [w2648]
                frame #0 {
                  # "w (rad/s)"
                  # "t (s)"
                  n1688 = Divide(x=w2531, y=i64 1000) -> (x/y=w2507:dbl)
                  n1689 = local read "BD 1 Frequency 2 (MHz)"() -> (w2509:dbl)
                  n1690 = Multiply(x="Osc. freq. (Hz)", y=6.283185307179586) -> (x*y=w2529:dbl)
                  n1691 = Multiply(x=w2507, y=w2532) -> (x*y=w2528:dbl)
                  n1692 = Multiply(x=w2529, y=w2528) -> (x*y=w2512:dbl)
                  n1693 = local read "BD 1 Frequency 1 (MHz)"() -> (w2517:dbl)
                  n1694 = case shown="True" w2515 {
                    tunnel: w2512 -> [w2538 w2555]
                    tunnel: w2517 -> [_ w2563]
                    tunnel: w2509 -> [_ w2564]
                    tunnel: [w2535 w2559] -> w2508
                    tunnel: [FALSE w2540] -> w2513
                    tunnel: [0.0 w2551] -> w2510
                    frame False {
                      n1695 = Sine(x=w2538) -> (sin(x)=w2536:dbl)
                      n1696 = Multiply(x=w2536, y="Osc. amp. (MHz)") -> (x*y=w2535:dbl)
                    }
                    frame True {
                      # "trap position goes from 0 to 1 (0 is when it is furthest away, 1 is when closest)\nso we want to test for tether only when farther away, or x < 1"
                      # "quit if taking too long"
                      # "oscillate the trap"
                      # "Test for tether"
                      n1697 = local read "Vec Mean of T1 T2"() -> (w2539:dbl[])
                      "Trigger Signal" <- w2539
                      n1698 = Cosine(x=w2555) -> (cos(x)=w2567:dbl)
                      n1699 = Subtract(x=w2564, y=w2563) -> (x-y=w2562:dbl)
                      n1700 = Decrement(x=w2567) -> (x-1=w2566:dbl)
                      n1701 = Subtract(x=w2562, y="Closest Delta (MHz)") -> (x-y=w2560:dbl)
                      n1702 = Divide(x=w2566, y=-2.0) -> (x/y=w2550:dbl)
                      n1703 = Greater?(x=w2539, y="Stop F (pN)") -> (0:w2557:bool[])
                      n1704 = Multiply(x=w2550, y=w2560) -> (x*y=w2559:dbl)
                      n1705 = Less?(x=w2550, y="Fish mask thresh") -> (x < y?=w2549:bool)
                      n1706 = Boolean To (0,1)(Boolean=w2549) -> (0, 1=w2547:i16)
                      n1707 = Multiply(x=w2547, y=w2539) -> (x*y=w2546:dbl[])
                      n1708 = Divide(x=w2555, y=6.283185307179586) -> (x/y=w2554:dbl)
                      n1709 = Round Toward +Infinity(x=w2554) -> (ceil(x): smallest int >= x=w2551:dbl)
                      "Attempts" <- w2551